vi "Controle_Manip_Main_GUI_WorkingBackup_211222.vi"() -> ()   [LabVIEW 2019] (continued)
                            n865 = control-ref of="N Step Power  Diode Current (A)"() -> (w1168:refnum<vi>)
                            n866 = control-ref of="End Power  Diod Current (A)"() -> (w1169:refnum<vi>)
                            n867 = control-ref of="Start Power Diod Current (A)"() -> (w1170:refnum<vi>)
                            n868 = property class="Bool (strict)"(reference=w1167, "Value"=FALSE) -> ()  [unwired: 1 in, 2 out]
                            n869 = control-ref of="Acquire fPow"() -> (w1174:refnum<vi>)
                            n870 = control-ref of="Save fPow"() -> (w1172:refnum<vi>)
                            n871 = Build Array(w1174, w1172, w1170, w1169, w1168) -> (w1173:refnum<vi>[])
                            n872 = call "Enable&Disable_Controls.vi"("Enum"=enum16{"Enabled", "Disabled", "Disabled&Grayed"}."Enabled", "References"=w1173) -> ()  [unwired: 1 in]
                            n873 = property on="Elapsed (s)" class="DigNum (strict)"("Visible"=FALSE) -> ()  [unwired: 2 in, 2 out]
                            n874 = local read "Auto< ?"() -> (w1162:bool)
                            n875 = control-ref of="Save fPow"() -> (w1164:refnum<vi>)
                            n876 = case shown="True" w1162 {
                              tunnel: [TRUE FALSE] -> w1161
                              frame False {
                              }
                              frame True {
                              }
                            }
                            n877 = control-ref of="MasterStop"() -> (w1159:refnum<vi>)
                            n878 = control-ref of="MasterPause"() -> (w1160:refnum<vi>)
                            n879 = control-ref of="ExperimentStopped?"() -> (w1158:refnum<vi>)
                            n880 = call "CheckStopAndReset.vi"("ExperimentStopped?"=w1158, "MasterStop"=w1159, "MasterPause"=w1160) -> ()
                            n881 = control-ref of="Acquire fPow"() -> (w1165:refnum<vi>)
                            n882 = property class="Bool (strict)"(reference=w1165, "Visible"=TRUE) -> ()  [unwired: 1 in, 2 out]
                            n883 = property class="Bool (strict)"(reference=w1164, "Visible"=w1161) -> ()  [unwired: 1 in, 2 out]
                            n884 = property on="CCD 2D Image Main" class="IntGraph (strict)"("Visible"=TRUE) -> ()  [unwired: 2 in, 2 out]
                            n885 = property on="CCD 1D Spectrum Main" class="XYGraph (strict)"("Visible"=FALSE) -> ()  [unwired: 2 in, 2 out]
                          }
                        }
                      }
                      frame "Fast Acq" {
                        n886 = stacked-sequence {
                          frame #0 {
                            w1177 = AcqMode."Spectrum" ("Acq Mode")
                            # "set port to CCD if not already"
                            n887 = property on="Acq Mode" class="Enum (strict)"() -> ("Value"=w1179:T3)  [unwired: 2 in, 2 out]
                            n888 = Not Equal?(x=w1179, y=w1177) -> (x != y?=w1178:bool)
                            n889 = case shown="True" w1178 {
                              tunnel: w1177 -> [_ w1181]
                              frame False {
                              }
                              frame True {
                                w1180 = T33 4 items=["None"=1, "SideEntrance"=2, "FrontEntrance"=3, "SideExit"=5, "FrontExit"=4] ("Exit Port Location")
                                n890 = local read "LightField Automation error out"() -> (w1191:errorcluster)
                                n891 = local read "LightField Automation out"() -> (w1190:refnum<class "LightField Automation.lvclass">)
                                n892 = property on="Acq Mode" class="Enum (strict)"("Value"=w1181) -> ()  [unwired: 2 in, 2 out]
                                n893 = call "spec_SetOpticalExitPort.vi"("error in (no error)"=w1191, "Exit Port Location"=w1180, "LightField Automation in"=w1190) -> ("error out"=w1183:errorcluster, "LightField Automation out"=w1182:refnum<class "LightField Automation.lvclass">)  [unwired: 7 in]
                                n894 = call "spec_GetCenterWavelength.vi"("error in (no error)"=w1183, "LightField Automation in"=w1182) -> ("error out"=w1186:errorcluster, "Center Wavelength"=w1184:dbl, "LightField Automation out"=w1185:refnum<class "LightField Automation.lvclass">)  [unwired: 7 in]
                                n895 = local write "Exit mirror"(w1180) -> ()
                                n896 = local write "Center Wavelength (nm)"(w1184) -> ()
                                n897 = call "spec_getCalibration.vi"("error in (no error)"=w1186, "LightField Automation in"=w1185) -> ("error out"=w1189:errorcluster, "ColumnCalibration"=w1187:dbl[], "LightField Automation out"=w1188:refnum<class "LightField Automation.lvclass">)  [unwired: 7 in]
                                n898 = local write "Wavelength calibration"(w1187) -> ()
                                n899 = local write "LightField Automation error out"(w1189) -> ()
                                n900 = local write "LightField Automation out"(w1188) -> ()
                              }
                            }
                          }
                          frame #1 {
                            # "background if none"
                            n901 = local read "Background taken?"() -> (w1192:bool)
                            n902 = case shown="False" w1192 {
                              frame False {
                                n903 = stacked-sequence {
                                tunnel: [_ _ w1238] -> w1193
                                frame #0 {
                                n904 = property on="CCD 1D Spectrum Main" class="XYGraph (strict)"("YScale.Offset"=0.0 ("Y Scale.Offset and Multiplier:Offset")) -> ()  [unwired: 2 in, 2 out]
                                }
                                frame #1 {
                                # "make sure shutter is closed"
                                n905 = local read "KCube Shutter On?"() -> (w1224:bool)
                                n906 = control-ref of="Shutter Ctrls"() -> (w1228:refnum<vi>)
                                n907 = property class="Ring (strict)"(reference=w1228) -> ("Value"=w1227:u16)  [unwired: 1 in, 2 out]
                                n908 = control-ref of="KCube Shutter Device Reference"() -> (w1229:refnum<vi>)
                                n909 = Equal?(x=w1227, y=u16 0) -> (x = y?=w1225:bool)
                                n910 = case shown="False" w1225 {
                                tunnel: w1229 -> [w1232 _]
                                tunnel: w1228 -> [w1231 _]
                                tunnel: w1224 -> [w1230 _]
                                frame False {
                                n911 = call "Shutter.vi"("KCube Shutter Device Reference 2"=w1232, "Shutter Ctrls 2"=w1231, "Shutter on?"=w1230) -> ()
                                }
                                frame True {
                                }
                                }
                                }
                                frame #2 {
                                # "acquire"
                                n912 = local read "LightField Automation error out"() -> (w1236:errorcluster)
                                n913 = local read "LightField Automation out"() -> (w1237:refnum<class "LightField Automation.lvclass">)
                                n914 = local read "Accumulations"() -> (w1233:dbl)
                                n915 = call "LFA_Capture.vi"("error in (no error)"=w1236, "Frames"=w1233, "LightField Automation in"=w1237) -> ("error out"=w1235:errorcluster, "Data"=w1238:T26, "LightField Automation out"=w1234:refnum<class "LightField Automation.lvclass">)  [unwired: 6 in]
                                n916 = local write "LightField Automation error out"(w1235) -> ()
                                n917 = local write "LightField Automation out"(w1234) -> ()
                                }
                                }
                                n918 = local read "Acq Mode"() -> (w1194:T3)
                                n919 = case shown="\"Spectrum\", Default" w1194 {
                                selector: w1194 -> [w1195 w1213]
                                tunnel: w1193 -> [w1196 w1214]
                                frame "Spectrum", Default {
                                n920 = stacked-sequence {
                                tunnel: w1196 -> [_ w1207 _ _]
                                tunnel: w1195 -> [_ w1205 _ _]
                                frame #0 {
                                n921 = property on="CCD 2D Image Main" class="IntGraph (strict)"("Visible"=FALSE) -> ()  [unwired: 2 in, 2 out]
                                n922 = property on="CCD 1D Spectrum Main" class="XYGraph (strict)"("Visible"=TRUE) -> ()  [unwired: 2 in, 2 out]
                                }
                                frame #1 {
                                n923 = local read "Wavelength calibration"() -> (w1204:dbl[])
                                n924 = local read "CCD ROI"() -> (w1200:T20)
                                n925 = Divide(x=1239.842, y=w1204) -> (x/y=w1202:dbl[])
                                n926 = call "PrepareData4Graph.vi"("Wavelength nm"=w1202, "DataLF"=w1207, "CCD ROI"=w1200, "AcqMode"=w1205, "Data type"=T30."Spectre") -> ("Spectrum"=w1206:cluster{"Array 2":dbl[], "Array":dbl[]}, "PLInt out"=w1199:dbl[])  [unwired: 2 in, 2 out]
                                n927 = local write "CCD 1D Spectrum Main"(w1206) -> ()
                                n928 = local write "BackgroundSpec"(w1199) -> ()
                                }
                                frame #2 {
                                n929 = local read "BackgroundSpec"() -> (w1208:dbl[])
                                n930 = call-poly <vilib>:"Mean.vi"("X"=w1208) -> ("mean"=w1210:dbl)  [unwired: 1 out]
                                n931 = Negate(x=w1210) -> (-x=w1209:dbl)
                                n932 = property on="CCD 1D Spectrum Main" class="XYGraph (strict)"("YScale.Offset"=w1209) -> ()  [unwired: 2 in, 2 out]
                                }
                                frame #3 {
                                n933 = local write "Background taken?"(TRUE ("Background taken?")) -> ()
                                n934 = property on="Background substract" class="Enum (strict)"("Value"=enum16{"None", "Shutter"}."None" ("Background substract")) -> ()  [unwired: 2 in, 2 out]
                                }
                                }
                                }
                                frame "Image" {
                                n935 = stacked-sequence {
                                tunnel: w1214 -> [_ w1222]
                                tunnel: w1213 -> [_ w1220]
                                frame #0 {
                                n936 = property on="CCD 1D Spectrum Main" class="XYGraph (strict)"("Visible"=FALSE) -> ()  [unwired: 2 in, 2 out]
                                n937 = property on="CCD 2D Image Main" class="IntGraph (strict)"("Visible"=TRUE) -> ()  [unwired: 2 in, 2 out]
                                }
                                frame #1 {
                                n938 = local read "Wavelength calibration"() -> (w1221:dbl[])
                                n939 = local read "CCD ROI"() -> (w1217:T20)
                                n940 = call "PrepareData4Graph.vi"("Wavelength nm"=w1221, "DataLF"=w1222, "CCD ROI"=w1217, "AcqMode"=w1220, "Data type"=T30."Spectre") -> ("Intensity Graph"=w1219:dbl[][])  [unwired: 2 in, 3 out]
                                n941 = local write "CCD 2D Image Main"(w1219) -> ()
                                }
                                }
                                }
                                }
                              }
                              frame True {
                              }
                            }
                          }
                          frame #2 {
                            # "\"measurement\""
                            n942 = stacked-sequence {
                              frame #0 {
                                # "open shutter if closed"
                                n943 = control-ref of="Shutter Ctrls"() -> (w1240:refnum<vi>)
                                n944 = property class="Ring (strict)"(reference=w1240) -> ("Value"=w1242:u16)  [unwired: 1 in, 2 out]
                                n945 = local read "KCube Shutter On?"() -> (w1245:bool)
                                n946 = control-ref of="KCube Shutter Device Reference"() -> (w1241:refnum<vi>)
                                n947 = property on="Experiment Graph Controls" class="TabCtl (strict)"("Value"=T25."Spectrum" ("Experiment Graph Controls")) -> ()  [unwired: 2 in, 2 out]
                                n948 = Equal?(x=w1242, y=u16 0) -> (x = y?=w1244:bool)
                                n949 = case shown="True" w1244 {
                                tunnel: w1241 -> [_ w1248]
                                tunnel: w1240 -> [_ w1247]
                                tunnel: w1245 -> [_ w1246]
                                frame False {
                                }
                                frame True {
                                n950 = call "Shutter.vi"("KCube Shutter Device Reference 2"=w1248, "Shutter Ctrls 2"=w1247, "Shutter on?"=w1246) -> ()
                                }
                                }
                              }
                              frame #1 {
                                # "set CCD ROI and acquire"
                                n951 = local read "LightField Automation error out"() -> (w1256:errorcluster)
                                n952 = local read "LightField Automation out"() -> (w1257:refnum<class "LightField Automation.lvclass">)
                                n953 = local read "CCD ROI"() -> (w1255:T20)
                                n954 = local read "Accumulations"() -> (w1252:dbl)
                                n955 = call "Adv_SetROI.vi"("error in (no error)"=w1256, "ROI"=w1255, "LightField Automation in"=w1257) -> ("error out"=w1253:errorcluster, "LightField Automation out"=w1254:refnum<class "LightField Automation.lvclass">)  [unwired: 7 in]
                                n956 = call "LFA_Capture.vi"("error in (no error)"=w1253, "Frames"=w1252, "LightField Automation in"=w1254) -> ("error out"=w1250:errorcluster, "Data"=w1249:T26, "LightField Automation out"=w1251:refnum<class "LightField Automation.lvclass">)  [unwired: 6 in]
                                n957 = local write "LightField Automation out"(w1251) -> ()
                                n958 = local write "LightField Automation error out"(w1250) -> ()
                                n959 = local write "Data"(w1249) -> ()
                              }
                              frame #2 {
                                # "close shutter"
                                n960 = local read "KCube Shutter On?"() -> (w1260:bool)
                                n961 = control-ref of="KCube Shutter Device Reference"() -> (w1259:refnum<vi>)
                                n962 = control-ref of="Shutter Ctrls"() -> (w1258:refnum<vi>)
                                n963 = call "Shutter.vi"("KCube Shutter Device Reference 2"=w1259, "Shutter Ctrls 2"=w1258, "Shutter on?"=w1260) -> ()
                              }
                              frame #3 {
                                # "Show data accordingly"
                                n964 = local read "Acq Mode"() -> (w1262:T3)
                                n965 = local read "Data"() -> (w1261:T26)
                                n966 = case shown="\"Spectrum\", Default" w1262 {
                                selector: w1262 -> [w1263 w1282]
                                tunnel: w1261 -> [w1264 w1283]
                                frame "Spectrum", Default {
                                n967 = stacked-sequence {
                                tunnel: w1264 -> [_ w1280 _]
                                tunnel: w1263 -> [_ w1278 _]
                                frame #0 {
                                n968 = property on="CCD 1D Spectrum Main" class="XYGraph (strict)"("Visible"=TRUE) -> ()  [unwired: 2 in, 2 out]
                                n969 = property on="CCD 2D Image Main" class="IntGraph (strict)"("Visible"=FALSE) -> ()  [unwired: 2 in, 2 out]
                                }
                                frame #1 {
                                n970 = local read "Wavelength calibration"() -> (w1277:dbl[])
                                n971 = local read "CCD ROI"() -> (w1273:T20)
                                n972 = Divide(x=1239.842, y=w1277) -> (x/y=w1275:dbl[])
                                n973 = call "PrepareData4Graph.vi"("Wavelength nm"=w1275, "DataLF"=w1280, "CCD ROI"=w1273, "AcqMode"=w1278, "Data type"=T30."Spectre") -> ("Spectrum"=w1279:cluster{"Array 2":dbl[], "Array":dbl[]}, "PLInt out"=w1272:dbl[])  [unwired: 2 in, 2 out]
                                n974 = local read "Excitation Power (uW)"() -> (w1269:dbl)
                                n975 = local write "CCD 1D Spectrum Main"(w1279) -> ()
                                n976 = local read "Acq Time (ms)"() -> (w1270:dbl)
                                n977 = local read "BackgroundSpec"() -> (w1268:dbl[])
                                n978 = local read "Display Mode"() -> (w1267:u16)
                                n979 = control-ref of="Cnts"() -> (w1271:refnum<vi>)
                                n980 = call "2Cnts.vi"("Array Background"=w1268, "Pow W"=w1269, "AcqTime ms"=w1270, "Cnts Ref"=w1271, "Display Mode"=w1267, "Array"=w1272) -> ()  [unwired: 1 out]
                                }
                                frame #2 {
                                n981 = property on="Full scale" class="Bool (strict)"("Val(Sgnl)"=TRUE ("Value (Signaling)")) -> ()  [unwired: 2 in, 2 out]
                                }
                                }
                                }
                                frame "Image" {
                                n982 = stacked-sequence {
                                tunnel: w1283 -> [_ w1291]
                                tunnel: w1282 -> [_ w1289]
                                frame #0 {
                                n983 = property on="CCD 1D Spectrum Main" class="XYGraph (strict)"("Visible"=FALSE) -> ()  [unwired: 2 in, 2 out]
                                n984 = property on="CCD 2D Image Main" class="IntGraph (strict)"("Visible"=TRUE) -> ()  [unwired: 2 in, 2 out]
                                }
                                frame #1 {
                                n985 = local read "Wavelength calibration"() -> (w1290:dbl[])
                                n986 = local read "CCD ROI"() -> (w1286:T20)
                                n987 = call "PrepareData4Graph.vi"("Wavelength nm"=w1290, "DataLF"=w1291, "CCD ROI"=w1286, "AcqMode"=w1289, "Data type"=T30."Spectre") -> ("Intensity Graph"=w1288:dbl[][])  [unwired: 2 in, 3 out]
                                n988 = local write "CCD 2D Image Main"(w1288) -> ()
                                }
                                }
                                }
                                }
                              }
                            }
                          }
                        }
                      }
                      frame "Acquire Custom Diode Spectrum" {
                        n989 = stacked-sequence {
                          frame #0 {
                            # "change exit slit to APD if needed"
                            n990 = local read "Spectrum Custom Mode"() -> (w1293:u16)
                            n991 = case shown="3" w1293 {
                              frame 0, Default {
                                n992 = control-ref of="Accumulations"() -> (w1300:refnum<vi>)
                                n993 = control-ref of="CCD ROI"() -> (w1301:refnum<vi>)
                                n994 = control-ref of="Exposure Time (ms)"() -> (w1302:refnum<vi>)
                                n995 = stacked-sequence {
                                tunnel: u16 5 ("NewVal") -> [w1304 w1309 _]
                                tunnel: [_ w1308 _] -> w1298
                                tunnel: [_ w1307 _] -> w1297
                                frame #0 {
                                n996 = control-ref of="Exit mirror"() -> (w1303:refnum<vi>)
                                n997 = property class="Ring (strict)"(reference=w1303, "Value"=w1304) -> ()  [unwired: 1 in, 2 out]
                                n998 = Build Array(w1303) -> (w1306:refnum<vi>[])
                                n999 = call "Enable&Disable_Controls.vi"("Enum"=enum16{"Enabled", "Disabled", "Disabled&Grayed"}."Disabled&Grayed", "References"=w1306) -> ()  [unwired: 1 in]
                                }
                                frame #1 {
                                n1000 = local read "LightField Automation error out"() -> (w1317:errorcluster)
                                n1001 = case shown="4, Default" w1309 {
                                tunnel: [enum16{"Enabled", "Disabled", "Disabled&Grayed"}."Disabled&Grayed" ("Enum") enum16{"Enabled", "Disabled", "Disabled&Grayed"}."Enabled" ("Enum")] -> w1308
                                tunnel: [AcqMode."APD 1" ("Acq Mode") AcqMode."Spectrum" ("Acq Mode")] -> w1307
                                frame 5 {
                                }
                                frame 4, Default {
                                }
                                }
                                n1002 = local read "LightField Automation out"() -> (w1316:refnum<class "LightField Automation.lvclass">)
                                n1003 = call "spec_GetOpticalExitPort.vi"("error in (no error)"=w1317, "LightField Automation in"=w1316) -> ("error out"=w1314:errorcluster, "Exit Port Location"=w1313:T33, "LightField Automation out"=w1315:refnum<class "LightField Automation.lvclass">)  [unwired: 7 in]
                                n1004 = Equal?(x=w1313, y=w1309) -> (x = y?=w1312:bool)
                                n1005 = case shown="False" w1312 {
                                tunnel: w1315 -> [w1338 w1340]
                                tunnel: w1314 -> [w1337 w1339]
                                tunnel: w1309 -> [w1336 _]
                                tunnel: [w1329 w1340] -> w1311
                                tunnel: [w1328 w1339] -> w1310
                                frame False {
                                n1006 = call "spec_SetOpticalExitPort.vi"("error in (no error)"=w1337, "Exit Port Location"=w1336, "LightField Automation in"=w1338) -> ("error out"=w1331:errorcluster, "LightField Automation out"=w1330:refnum<class "LightField Automation.lvclass">)  [unwired: 7 in]
                                n1007 = call "spec_GetCenterWavelength.vi"("error in (no error)"=w1331, "LightField Automation in"=w1330) -> ("error out"=w1334:errorcluster, "Center Wavelength"=w1332:dbl, "LightField Automation out"=w1333:refnum<class "LightField Automation.lvclass">)  [unwired: 7 in]
                                n1008 = local write "Center Wavelength (nm)"(w1332) -> ()
                                n1009 = call "spec_getCalibration.vi"("error in (no error)"=w1334, "LightField Automation in"=w1333) -> ("error out"=w1328:errorcluster, "ColumnCalibration"=w1335:dbl[], "LightField Automation out"=w1329:refnum<class "LightField Automation.lvclass">)  [unwired: 7 in]
                                n1010 = local write "Wavelength calibration"(w1335) -> ()
                                n1011 = property on="Exit mirror" class="Ring (strict)"() -> ("RingText.Text"=w1324:string)  [unwired: 2 in, 2 out]
                                n1012 = local read "Log file"() -> (w1327:string)
                                n1013 = Concatenate Strings("Exit mirror set to " ("Add to log file"), w1324) -> (w1325:string)
                                n1014 = call "Write2LogFile.vi"("Add to log file"=w1325, "Log file before"=w1327, "Checkbox"=FALSE) -> ("Log file after"=w1326:string)
                                n1015 = local write "Log file"(w1326) -> ()
                                }
                                frame True {
                                }
                                }
                                n1016 = local write "LightField Automation error out"(w1310) -> ()
                                n1017 = local write "LightField Automation out"(w1311) -> ()
                                }
                                frame #2 {
                                n1018 = control-ref of="Exit mirror"() -> (w1343:refnum<vi>)
                                n1019 = Build Array(w1343) -> (w1342:refnum<vi>[])
                                n1020 = call "Enable&Disable_Controls.vi"("Enum"=enum16{"Enabled", "Disabled", "Disabled&Grayed"}."Enabled", "References"=w1342) -> ()  [unwired: 1 in]
                                }
                                }
                                n1021 = Build Array(w1300, w1301, w1302) -> (w1299:refnum<vi>[])
                                n1022 = call "Enable&Disable_Controls.vi"("Enum"=w1298, "References"=w1299) -> ()  [unwired: 1 in]
                                n1023 = property on="Acq Mode" class="Enum (strict)"("Value"=w1297) -> ()  [unwired: 2 in, 2 out]
                              }
                              frame 1 {
                                n1024 = control-ref of="Accumulations"() -> (w1348:refnum<vi>)
                                n1025 = control-ref of="CCD ROI"() -> (w1349:refnum<vi>)
                                n1026 = control-ref of="Exposure Time (ms)"() -> (w1350:refnum<vi>)
                                n1027 = stacked-sequence {
                                tunnel: u16 5 ("NewVal") -> [w1352 w1357 _]
                                tunnel: [_ w1356 _] -> w1346
                                tunnel: [_ w1355 _] -> w1345
                                frame #0 {
                                n1028 = control-ref of="Exit mirror"() -> (w1351:refnum<vi>)
                                n1029 = property class="Ring (strict)"(reference=w1351, "Value"=w1352) -> ()  [unwired: 1 in, 2 out]
                                n1030 = Build Array(w1351) -> (w1354:refnum<vi>[])
                                n1031 = call "Enable&Disable_Controls.vi"("Enum"=enum16{"Enabled", "Disabled", "Disabled&Grayed"}."Disabled&Grayed", "References"=w1354) -> ()  [unwired: 1 in]
                                }
                                frame #1 {
                                n1032 = local read "LightField Automation error out"() -> (w1365:errorcluster)
                                n1033 = case shown="5" w1357 {
                                tunnel: [enum16{"Enabled", "Disabled", "Disabled&Grayed"}."Disabled&Grayed" ("Enum") enum16{"Enabled", "Disabled", "Disabled&Grayed"}."Enabled" ("Enum")] -> w1356
                                tunnel: [AcqMode."APD 1" ("Acq Mode") AcqMode."Spectrum" ("Acq Mode")] -> w1355
                                frame 5 {
                                }
                                frame 4, Default {
                                }
                                }
                                n1034 = local read "LightField Automation out"() -> (w1364:refnum<class "LightField Automation.lvclass">)
                                n1035 = call "spec_GetOpticalExitPort.vi"("error in (no error)"=w1365, "LightField Automation in"=w1364) -> ("error out"=w1362:errorcluster, "Exit Port Location"=w1361:T33, "LightField Automation out"=w1363:refnum<class "LightField Automation.lvclass">)  [unwired: 7 in]
                                n1036 = Equal?(x=w1361, y=w1357) -> (x = y?=w1360:bool)
                                n1037 = case shown="False" w1360 {
                                tunnel: w1363 -> [w1386 w1388]
                                tunnel: w1362 -> [w1385 w1387]
                                tunnel: w1357 -> [w1384 _]
                                tunnel: [w1377 w1388] -> w1359
                                tunnel: [w1376 w1387] -> w1358
                                frame False {
                                n1038 = call "spec_SetOpticalExitPort.vi"("error in (no error)"=w1385, "Exit Port Location"=w1384, "LightField Automation in"=w1386) -> ("error out"=w1379:errorcluster, "LightField Automation out"=w1378:refnum<class "LightField Automation.lvclass">)  [unwired: 7 in]
                                n1039 = call "spec_GetCenterWavelength.vi"("error in (no error)"=w1379, "LightField Automation in"=w1378) -> ("error out"=w1382:errorcluster, "Center Wavelength"=w1380:dbl, "LightField Automation out"=w1381:refnum<class "LightField Automation.lvclass">)  [unwired: 7 in]
                                n1040 = local write "Center Wavelength (nm)"(w1380) -> ()
                                n1041 = call "spec_getCalibration.vi"("error in (no error)"=w1382, "LightField Automation in"=w1381) -> ("error out"=w1376:errorcluster, "ColumnCalibration"=w1383:dbl[], "LightField Automation out"=w1377:refnum<class "LightField Automation.lvclass">)  [unwired: 7 in]
                                n1042 = local write "Wavelength calibration"(w1383) -> ()
                                n1043 = property on="Exit mirror" class="Ring (strict)"() -> ("RingText.Text"=w1372:string)  [unwired: 2 in, 2 out]
                                n1044 = local read "Log file"() -> (w1375:string)
                                n1045 = Concatenate Strings("Exit mirror set to " ("Add to log file"), w1372) -> (w1373:string)
                                n1046 = call "Write2LogFile.vi"("Add to log file"=w1373, "Log file before"=w1375, "Checkbox"=FALSE) -> ("Log file after"=w1374:string)
                                n1047 = local write "Log file"(w1374) -> ()
                                }
                                frame True {
                                }
                                }
                                n1048 = local write "LightField Automation error out"(w1358) -> ()
                                n1049 = local write "LightField Automation out"(w1359) -> ()
                                }
                                frame #2 {
                                n1050 = control-ref of="Exit mirror"() -> (w1391:refnum<vi>)
                                n1051 = Build Array(w1391) -> (w1390:refnum<vi>[])
                                n1052 = call "Enable&Disable_Controls.vi"("Enum"=enum16{"Enabled", "Disabled", "Disabled&Grayed"}."Enabled", "References"=w1390) -> ()  [unwired: 1 in]
                                }
                                }
                                n1053 = Build Array(w1348, w1349, w1350) -> (w1347:refnum<vi>[])
                                n1054 = call "Enable&Disable_Controls.vi"("Enum"=w1346, "References"=w1347) -> ()  [unwired: 1 in]
                                n1055 = property on="Acq Mode" class="Enum (strict)"("Value"=w1345) -> ()  [unwired: 2 in, 2 out]
                              }
                              frame 3 {
                                n1056 = control-ref of="Accumulations"() -> (w1396:refnum<vi>)
                                n1057 = control-ref of="CCD ROI"() -> (w1397:refnum<vi>)
                                n1058 = control-ref of="Exposure Time (ms)"() -> (w1398:refnum<vi>)
                                n1059 = stacked-sequence {
                                tunnel: u16 5 ("NewVal") -> [w1400 w1405 _]
                                tunnel: [_ w1404 _] -> w1394
                                tunnel: [_ w1403 _] -> w1393
                                frame #0 {
                                n1060 = control-ref of="Exit mirror"() -> (w1399:refnum<vi>)
                                n1061 = property class="Ring (strict)"(reference=w1399, "Value"=w1400) -> ()  [unwired: 1 in, 2 out]
                                n1062 = Build Array(w1399) -> (w1402:refnum<vi>[])
                                n1063 = call "Enable&Disable_Controls.vi"("Enum"=enum16{"Enabled", "Disabled", "Disabled&Grayed"}."Disabled&Grayed", "References"=w1402) -> ()  [unwired: 1 in]
                                }
                                frame #1 {
                                n1064 = local read "LightField Automation error out"() -> (w1413:errorcluster)
                                n1065 = case shown="4, Default" w1405 {
                                tunnel: [enum16{"Enabled", "Disabled", "Disabled&Grayed"}."Disabled&Grayed" ("Enum") enum16{"Enabled", "Disabled", "Disabled&Grayed"}."Enabled" ("Enum")] -> w1404
                                tunnel: [AcqMode."APD 1+2" ("Acq Mode") AcqMode."Spectrum" ("Acq Mode")] -> w1403
                                frame 5 {
                                }
                                frame 4, Default {
                                }
                                }
                                n1066 = local read "LightField Automation out"() -> (w1412:refnum<class "LightField Automation.lvclass">)
                                n1067 = call "spec_GetOpticalExitPort.vi"("error in (no error)"=w1413, "LightField Automation in"=w1412) -> ("error out"=w1410:errorcluster, "Exit Port Location"=w1409:T33, "LightField Automation out"=w1411:refnum<class "LightField Automation.lvclass">)  [unwired: 7 in]
                                n1068 = Equal?(x=w1409, y=w1405) -> (x = y?=w1408:bool)
                                n1069 = case shown="False" w1408 {
                                tunnel: w1411 -> [w1434 w1436]
                                tunnel: w1410 -> [w1433 w1435]
                                tunnel: w1405 -> [w1432 _]
                                tunnel: [w1425 w1436] -> w1407
                                tunnel: [w1424 w1435] -> w1406
                                frame False {
                                n1070 = call "spec_SetOpticalExitPort.vi"("error in (no error)"=w1433, "Exit Port Location"=w1432, "LightField Automation in"=w1434) -> ("error out"=w1427:errorcluster, "LightField Automation out"=w1426:refnum<class "LightField Automation.lvclass">)  [unwired: 7 in]
                                n1071 = call "spec_GetCenterWavelength.vi"("error in (no error)"=w1427, "LightField Automation in"=w1426) -> ("error out"=w1430:errorcluster, "Center Wavelength"=w1428:dbl, "LightField Automation out"=w1429:refnum<class "LightField Automation.lvclass">)  [unwired: 7 in]
                                n1072 = local write "Center Wavelength (nm)"(w1428) -> ()
                                n1073 = call "spec_getCalibration.vi"("error in (no error)"=w1430, "LightField Automation in"=w1429) -> ("error out"=w1424:errorcluster, "ColumnCalibration"=w1431:dbl[], "LightField Automation out"=w1425:refnum<class "LightField Automation.lvclass">)  [unwired: 7 in]
                                n1074 = local write "Wavelength calibration"(w1431) -> ()
                                n1075 = property on="Exit mirror" class="Ring (strict)"() -> ("RingText.Text"=w1420:string)  [unwired: 2 in, 2 out]
                                n1076 = local read "Log file"() -> (w1423:string)
                                n1077 = Concatenate Strings("Exit mirror set to " ("Add to log file"), w1420) -> (w1421:string)
                                n1078 = call "Write2LogFile.vi"("Add to log file"=w1421, "Log file before"=w1423, "Checkbox"=FALSE) -> ("Log file after"=w1422:string)
                                n1079 = local write "Log file"(w1422) -> ()
                                }
                                frame True {
                                }
                                }
                                n1080 = local write "LightField Automation error out"(w1406) -> ()
                                n1081 = local write "LightField Automation out"(w1407) -> ()
                                }
                                frame #2 {
                                n1082 = control-ref of="Exit mirror"() -> (w1439:refnum<vi>)
                                n1083 = Build Array(w1439) -> (w1438:refnum<vi>[])
                                n1084 = call "Enable&Disable_Controls.vi"("Enum"=enum16{"Enabled", "Disabled", "Disabled&Grayed"}."Enabled", "References"=w1438) -> ()  [unwired: 1 in]
                                }
                                }
                                n1085 = Build Array(w1396, w1397, w1398) -> (w1395:refnum<vi>[])
                                n1086 = call "Enable&Disable_Controls.vi"("Enum"=w1394, "References"=w1395) -> ()  [unwired: 1 in]
                                n1087 = property on="Acq Mode" class="Enum (strict)"("Value"=w1393) -> ()  [unwired: 2 in, 2 out]
                              }
                              frame 2 {
                                n1088 = property on="Acq Mode" class="Enum (strict)"("Value"=AcqMode."APD 2" ("Acq Mode")) -> ()  [unwired: 2 in, 2 out]
                              }
                              frame 4 {
                                n1089 = property on="Acq Mode" class="Enum (strict)"("Value"=AcqMode."APD 2" ("Acq Mode")) -> ()  [unwired: 2 in, 2 out]
                              }
                            }
                            n1090 = local read "Scan Spectrum Cust Params"() -> (w1295:refnum<vi>[])
                            n1091 = call "Enable&Disable_Controls.vi"("Enum"=enum16{"Enabled", "Disabled", "Disabled&Grayed"}."Disabled&Grayed", "References"=w1295) -> ()  [unwired: 1 in]
                            n1092 = property on="Experiment Graph Controls" class="TabCtl (strict)"("Value"=T25."Spectrum" ("Experiment Graph Controls")) -> ()  [unwired: 2 in, 2 out]
                          }
                          frame #1 {
                            n1093 = local read "Spectrum Step Wavelength (nm)"() -> (w1449:dbl)
                            n1094 = local read "Spectrum End Wavelength (nm)"() -> (w1448:dbl)
                            n1095 = local read "Spectrum Start Wavelength (nm)"() -> (w1450:dbl)
                            n1096 = local read "Spectrum Custom Mode"() -> (w1447:u16)
                            n1097 = local read "KCube Shutter On?"() -> (w1446:bool)
                            n1098 = local read "Acq Time (ms)"() -> (w1445:dbl)
                            n1099 = Bundle("Acq Time (ms)"=w1445, "Spectrum Start Wavelength (nm)"=w1450, "Spectrum Step Wavelength (nm)"=w1449, "Spectrum End Wavelength (nm)"=w1448, "Spectrum Custom Mode"=w1447, "KCube Shutter On?"=w1446) -> (→"Scan Spectrum Cust Exp Params":T18)  [unwired: 1 in]
                            n1100 = control-ref of="MasterStop"() -> (w1443:refnum<vi>)
                            n1101 = property class="Bool (strict)"(reference=w1443, "Visible"=TRUE) -> ()  [unwired: 1 in, 2 out]
                          }
                          frame #2 {
                            n1102 = local read "Spectrum Custom Mode"() -> (w1451:u16)
                            n1103 = case shown="1" w1451 {
                              frame 0, Default {
                                # "PD1 \nScan monochromator SpectraPro HRS with photodiode at APD exit slit"
                                n1104 = control-ref of="Scan Main Progess Bar"() -> (w1455:refnum<vi>)
                                n1105 = local read "LightField Automation out"() -> (w1467:refnum<class "LightField Automation.lvclass">)
                                n1106 = local read "Photodiode handle out"() -> (w1466:refnum<visa-resource-name>)
                                n1107 = local read "LightField Automation error out"() -> (w1464:errorcluster)
                                n1108 = local read "Photodiode error out"() -> (w1465:errorcluster)
                                n1109 = control-ref of="CCD 1D Spectrum Main"() -> (w1463:refnum<vi>)
                                n1110 = control-ref of="Center Wavelength (nm)"() -> (w1461:refnum<vi>)
                                n1111 = control-ref of="Stop Spectrum Custom"() -> ()  [unwired: 1 out]
                                n1112 = control-ref of="Excitation Power (uW)"() -> (w1456:refnum<vi>)
                                n1113 = local read "Scan Spectrum Cust Exp Params"() -> (w1462:T18)
                                n1114 = control-ref of="MasterStop"() -> (w1452:refnum<vi>)
                                n1115 = call "CustomSpectrum.vi"("LightField Automation"=w1467, "Photodiode handle out"=w1466, "Stop Spectrum Custom"=w1452, "Photodiode error out"=w1465, "LightField Automation error"=w1464, "CCD 1D Spectrum Main"=w1463, "Center Wavelength (nm)"=w1461, "Scan Spectrum Progess Bar"=w1455, "Excitation Power (uW)"=w1456, "Scan Spectrum Cust Exp Params 2"=w1462) -> ("WLs"=w1454:dbl[], "PL"=w1453:dbl[], "LFA Out"=w1460:refnum<class "LightField Automation.lvclass">, "PD Out"=w1459:refnum<visa-resource-name>, "PD Error Our"=w1458:errorcluster, "LFA Error Out"=w1457:errorcluster)  [unwired: 3 in, 1 out]
                                n1116 = local write "Data PL Custom Diode Spectrum"(w1453) -> ()
                                n1117 = local write "Wavelength calibration"(w1454) -> ()
                                n1118 = local write "LightField Automation out"(w1460) -> ()
                                n1119 = local write "Photodiode handle out"(w1459) -> ()
                                n1120 = local write "LightField Automation error out"(w1457) -> ()
                                n1121 = local write "Photodiode error out"(w1458) -> ()
                              }
                              frame 1 {
                                # "APD1 Scan monochromator SpectraPro HRS and acquire APD 1"
                                n1122 = stacked-sequence {
                                frame #0 {
                                n1123 = property on="Save Custom Diode Spectrum" class="Bool (strict)"("Visible"=FALSE) -> ()  [unwired: 2 in, 2 out]
                                n1124 = local read "KCube Shutter On?"() -> (w1472:bool)
                                n1125 = control-ref of="Shutter Ctrls"() -> (w1473:refnum<vi>)
                                n1126 = control-ref of="KCube Shutter Device Reference"() -> (w1474:refnum<vi>)
                                n1127 = call "Shutter.vi"("KCube Shutter Device Reference 2"=w1474, "Shutter Ctrls 2"=w1473, "Shutter on?"=w1472) -> ()
                                n1128 = property on="CCD 1D Spectrum Main" class="XYGraph (strict)"("YScale.Offset"=0.0 ("Y Scale.Offset and Multiplier:Offset"), "YScale.Minimum"=0.0 ("Y Scale.Range:Minimum")) -> ()  [unwired: 2 in, 2 out]
                                n1129 = property on="Elapsed (s)" class="DigNum (strict)"("Visible"=TRUE) -> ()  [unwired: 2 in, 2 out]
                                }
                                frame #1 {
                                n1130 = local read "PH_Init_Data"() -> (w1486:T11)
                                n1131 = local read "PH_Settings_Params"() -> (w1485:T10)
                                n1132 = Unbundle By Name(w1486) -> ("Deviceindex"=w1483:i32)
                                n1133 = local read "PH_CFD1 level"() -> (w1480:i32)
                                n1134 = local read "PH_CFD1 zero X"() -> (w1479:i32)
                                n1135 = local read "Acq Time (ms)"() -> (w1476:dbl)
                                n1136 = local read "PH_Range No."() -> (w1478:i32)
                                n1137 = local read "PH_CFD0 level"() -> (w1482:i32)
                                n1138 = local read "PH_CFD0 zero X"() -> (w1481:i32)
                                n1139 = local read "PH_SyncDiv"() -> (w1484:enum16{"1", "2", "4", "8"})
                                n1140 = Bundle By Name(cluster=w1485, "SyncDiv"=w1484, "DeviceIndex"=w1483, "CFD0 level"=w1482, "CFD0 zero X"=w1481, "CFD1 level"=w1480, "CFD1 zero X"=w1479, "Range No."=w1478, "StopOnOverflow"=TRUE, "AcqTime (ms)"=w1476) -> (w1475:T10)
                                n1141 = local write "PH_Settings_Params"(w1475) -> ()
                                }
                                frame #2 {
                                n1142 = local read "LightField Automation error out"() -> (w1495:errorcluster)
                                n1143 = local read "Scan Spectrum Cust Exp Params"() -> (w1494:T18)
                                n1144 = control-ref of="Center Wavelength (nm)"() -> (w1497:refnum<vi>)
                                n1145 = control-ref of="CCD 1D Spectrum Main"() -> (w1498:refnum<vi>)
                                n1146 = local read "LightField Automation out"() -> (w1496:refnum<class "LightField Automation.lvclass">)
                                n1147 = local read "PH_Settings_Params"() -> (w1492:T10)
                                n1148 = local read "PH_Init_Data"() -> (w1493:T11)
                                n1149 = control-ref of="Stop Spectrum Custom"() -> ()  [unwired: 1 out]
                                n1150 = control-ref of="Scan Main Progess Bar"() -> (w1499:refnum<vi>)
                                n1151 = control-ref of="MasterStop"() -> (w1487:refnum<vi>)
                                n1152 = call "CustomAPDSpectrum.vi"("LightField Automation"=w1496, "PH_Init_Data"=w1493, "PH_Settings_Params"=w1492, "Stop Spectrum Custom"=w1487, "LightField Automation error"=w1495, "CCD 1D Spectrum Main"=w1498, "Center Wavelength (nm)"=w1497, "Scan Spectrum Progess Bar"=w1499, "Scan Spectrum Cust Exp Params 2"=w1494) -> ("WLs"=w1489:dbl[], "LFA Out"=w1491:refnum<class "LightField Automation.lvclass">, "PL"=→"Data PL Custom Diode Spectrum":dbl[], "LFA Error Out"=w1490:errorcluster)  [unwired: 6 in, 1 out]
                                n1153 = local write "Wavelength calibration"(w1489) -> ()
                                n1154 = local write "LightField Automation error out"(w1490) -> ()
                                n1155 = local write "LightField Automation out"(w1491) -> ()
                                }
                                frame #3 {
                                n1156 = local read "KCube Shutter On?"() -> (w1505:bool)
                                n1157 = control-ref of="Shutter Ctrls"() -> (w1506:refnum<vi>)
                                n1158 = control-ref of="KCube Shutter Device Reference"() -> (w1507:refnum<vi>)
                                n1159 = call "Shutter.vi"("KCube Shutter Device Reference 2"=w1507, "Shutter Ctrls 2"=w1506, "Shutter on?"=w1505) -> ()
                                n1160 = property on="Full scale" class="Bool (strict)"("Val(Sgnl)"=TRUE ("Value (Signaling)")) -> ()  [unwired: 2 in, 2 out]
                                n1161 = property on="Elapsed (s)" class="DigNum (strict)"("Visible"=FALSE) -> ()  [unwired: 2 in, 2 out]
                                n1162 = local write "Background taken?"(FALSE ("Background taken?")) -> ()
                                n1163 = property on="CCD 1D Spectrum Main" class="XYGraph (strict)"("YScale.Offset"=0.0 ("Y Scale.Offset and Multiplier:Offset"), "YScale.Minimum"=0.0 ("Y Scale.Range:Minimum")) -> ()  [unwired: 2 in, 2 out]
                                }
                                }
                              }
                              frame 2 {
                                # "APD2 Scan monochromator iHR320 and acquire APD 2 // quick&dirty avant calib"
                                n1164 = stacked-sequence {
                                frame #0 {
                                w1508 = 0.0 ("Y Scale.Offset and Multiplier:Offset")
                                n1165 = property on="Elapsed (s)" class="DigNum (strict)"("Visible"=TRUE) -> ()  [unwired: 2 in, 2 out]
                                n1166 = property on="Save Custom Diode Spectrum" class="Bool (strict)"("Visible"=FALSE) -> ()  [unwired: 2 in, 2 out]
                                n1167 = local read "KCube Shutter On?"() -> (w1511:bool)
                                n1168 = control-ref of="Shutter Ctrls"() -> (w1512:refnum<vi>)
                                n1169 = control-ref of="KCube Shutter Device Reference"() -> (w1513:refnum<vi>)
                                n1170 = call "Shutter.vi"("KCube Shutter Device Reference 2"=w1513, "Shutter Ctrls 2"=w1512, "Shutter on?"=w1511) -> ()
                                n1171 = property on="CCD 1D Spectrum Main" class="XYGraph (strict)"("YScale.Offset"=w1508, "YScale.Minimum"=w1508) -> ()  [unwired: 2 in, 2 out]
                                }
                                frame #1 {
                                n1172 = local read "PH_Init_Data"() -> (w1524:T11)
                                n1173 = local read "PH_Settings_Params"() -> (w1525:T10)
                                n1174 = Unbundle By Name(w1524) -> ("Deviceindex"=w1522:i32)
                                n1175 = local read "PH_CFD1 level"() -> (w1519:i32)
                                n1176 = local read "PH_CFD1 zero X"() -> (w1518:i32)
                                n1177 = local read "Acq Time (ms)"() -> (w1516:dbl)
                                n1178 = local read "PH_Range No."() -> (w1517:i32)
                                n1179 = local read "PH_CFD0 level"() -> (w1521:i32)
                                n1180 = local read "PH_CFD0 zero X"() -> (w1520:i32)
                                n1181 = local read "PH_SyncDiv"() -> (w1523:enum16{"1", "2", "4", "8"})
                                n1182 = Bundle By Name(cluster=w1525, "SyncDiv"=w1523, "DeviceIndex"=w1522, "CFD0 level"=w1521, "CFD0 zero X"=w1520, "CFD1 level"=w1519, "CFD1 zero X"=w1518, "Range No."=w1517, "StopOnOverflow"=TRUE, "AcqTime (ms)"=w1516) -> (w1515:T10)
                                n1183 = local write "PH_Settings_Params"(w1515) -> ()
                                }
                                frame #2 {
                                n1184 = local read "Spectrum End Wavelength (nm)"() -> (w1533:dbl)
                                n1185 = local read "Spectrum Step Wavelength (nm)"() -> (w1527:dbl)
                                n1186 = local read "Spectrum Start Wavelength (nm)"() -> (w1531:dbl)
                                n1187 = Subtract(x=w1533, y=w1531) -> (x-y=w1535:dbl)
                                n1188 = Divide(x=w1535, y=w1527) -> (x/y=w1534:dbl)
                                n1189 = Increment(x=w1534) -> (x+1=w1532:dbl)
                                n1190 = for {
                                N: w1532 -> [_]
                                tunnel: w1527 -> [w1550]
                                tunnel: w1531 -> [w1549]
                                shift-right: [w1536] -> w1528
                                shift-left: dbl[] [] -> [w1544]
                                shift-right: [w1541] -> w1526
                                shift-left: dbl[] [] -> [w1545]
                                i -> [w1551]
                                stop <- w1539 stop-if-true
                                n1191 = control-ref of="MasterStop"() -> (w1538:refnum<vi>)
                                n1192 = control-ref of="Stop Spectrum Custom"() -> ()  [unwired: 1 out]
                                n1193 = Multiply(x=w1551, y=w1550) -> (x*y=w1548:dbl)
                                n1194 = Add(x=w1549, y=w1548) -> (x+y=w1540:dbl)
                                n1195 = local read "ESP300 COM Port"() -> (w1547:refnum<visa-resource-name>)
                                n1196 = stacked-sequence {
                                tunnel: w1540 -> [w1553 _ _]
                                tunnel: w1547 -> [w1561 _ _]
                                tunnel: [_ _ w1563] -> w1546
                                tunnel: w1545 -> [w1559 _ _]
                                tunnel: [w1558 _ _] -> w1541
                                frame #0 {
                                w1555 = u16 1 items=["Detection"=1, "Excitation"=2] ("HR mode")
                                n1197 = call "MotorWL2Pos.vi"("Mono2 Center WL"=w1553, "HR mode"=w1555) -> ("Mono2 Position"=w1557:dbl)
                                n1198 = control-ref of="Mono2 Motor Pos"() -> (w1560:refnum<vi>)
                                n1199 = control-ref of="Mono2 Wavelength (nm)"() -> (w1556:refnum<vi>)
                                n1200 = call "subVI_Mono2Go2Posv2.vi"("Mono2 Motor Pos"=w1560, "Mono2 Wavelength (nm)"=w1556, "HR mode"=w1555, "Postion (Unit)"=w1557, "ESP300 COM Port"=w1561) -> ()  [unwired: 2 out]
                                n1201 = Divide(x=1239.842, y=w1553) -> (x/y=w1552:dbl)
                                n1202 = Insert Into Array(array=w1559, new element=w1552) -> (w1558:dbl[])  [unwired: 1 in]
                                }
                                frame #1 {
                                n1203 = Wait (ms)(milliseconds to wait=u32 20) -> ()  [unwired: 1 out]
                                }
                                frame #2 {
                                n1204 = local read "PH_Settings_Params"() -> (w1564:T10)
                                n1205 = local read "PH_Init_Data"() -> (w1565:T11)
                                n1206 = Unbundle By Name(w1565) -> ("Initialization Error"=w1569:bool, "Calib Error"=w1568:bool, "Deviceindex"=w1567:i32)
                                n1207 = call "PH_Acq_ms.vi"("PH_Settings_Params"=w1564, "Deviceindex"=w1567, "Calib Error"=w1568, "Initialization Error"=w1569) -> ("CH1MeanRate"=w1563:dbl, "SyncMeanRate"=w1566:dbl)  [unwired: 1 out]
                                n1208 = Build Array(w1566, w1563) -> ()  [unwired: 1 out]
                                }
                                }
                                n1209 = property class="Bool (strict)"(reference=w1538) -> ("Value"=w1539:bool)  [unwired: 1 in, 2 out]
                                n1210 = control-ref of="CCD 1D Spectrum Main"() -> (w1543:refnum<vi>)
                                n1211 = Insert Into Array(array=w1544, new element=w1546) -> (w1536:dbl[])  [unwired: 1 in]
                                n1212 = call "myMaxAPDs.vi"("Array"=w1536) -> ("myMax"=w1537:dbl)
                                n1213 = Bundle(w1541, w1536) -> (w1542:cluster{dbl[], dbl[]})  [unwired: 1 in]
                                n1214 = property class="XYGraph (strict)"(reference=w1543, "Value"=w1542, "YScale.Maximum"=w1537) -> ()  [unwired: 1 in, 2 out]
                                }
                                n1215 = local write "Wavelength calibration"(w1526) -> ()
                                n1216 = local write "Data PL Custom Diode Spectrum"(w1528) -> ()
                                }
                                frame #3 {
                                n1217 = property on="Elapsed (s)" class="DigNum (strict)"("Visible"=FALSE) -> ()  [unwired: 2 in, 2 out]
                                n1218 = local read "KCube Shutter On?"() -> (w1575:bool)
                                n1219 = control-ref of="Shutter Ctrls"() -> (w1576:refnum<vi>)
                                n1220 = property on="CCD 1D Spectrum Main" class="XYGraph (strict)"("YScale.Offset"=0.0 ("Y Scale.Offset and Multiplier:Offset"), "YScale.Minimum"=0.0 ("Y Scale.Range:Minimum")) -> ()  [unwired: 2 in, 2 out]
                                n1221 = control-ref of="KCube Shutter Device Reference"() -> (w1577:refnum<vi>)
                                n1222 = call "Shutter.vi"("KCube Shutter Device Reference 2"=w1577, "Shutter Ctrls 2"=w1576, "Shutter on?"=w1575) -> ()
                                n1223 = local write "Background taken?"(FALSE ("Background taken?")) -> ()
                                n1224 = property on="Full scale" class="Bool (strict)"("Val(Sgnl)"=TRUE ("Value (Signaling)")) -> ()  [unwired: 2 in, 2 out]
                                }
                                }
                              }
                              frame 3 {
                                # "ADP1&2 Scan both monochromators synchronously and both APD outputs"
                              }
                              frame 4 {
                                # "PD2 Scan monochromator iHR320 with photodiode at APD exit slit"
                                n1225 = stacked-sequence {
                                frame #0 {
                                n1226 = property on="Elapsed (s)" class="DigNum (strict)"("Visible"=TRUE) -> ()  [unwired: 2 in, 2 out]
                                n1227 = property on="Save Custom Diode Spectrum" class="Bool (strict)"("Visible"=FALSE) -> ()  [unwired: 2 in, 2 out]
                                n1228 = local read "KCube Shutter On?"() -> (w1580:bool)
                                n1229 = control-ref of="Shutter Ctrls"() -> (w1581:refnum<vi>)
                                n1230 = control-ref of="KCube Shutter Device Reference"() -> (w1582:refnum<vi>)
                                n1231 = call "Shutter.vi"("KCube Shutter Device Reference 2"=w1582, "Shutter Ctrls 2"=w1581, "Shutter on?"=w1580) -> ()
                                }
                                frame #1 {
                                n1232 = local read "PH_Init_Data"() -> (w1593:T11)
                                n1233 = local read "PH_Settings_Params"() -> (w1594:T10)
                                n1234 = local read "PH_CFD1 level"() -> (w1588:i32)
                                n1235 = local read "PH_CFD1 zero X"() -> (w1587:i32)
                                n1236 = local read "Acq Time (ms)"() -> (w1585:dbl)
                                n1237 = local read "PH_Range No."() -> (w1586:i32)
                                n1238 = Unbundle By Name(w1593) -> ("Deviceindex"=w1591:i32)
                                n1239 = local read "PH_CFD0 level"() -> (w1590:i32)
                                n1240 = local read "PH_CFD0 zero X"() -> (w1589:i32)
                                n1241 = local read "PH_SyncDiv"() -> (w1592:enum16{"1", "2", "4", "8"})
                                n1242 = Bundle By Name(cluster=w1594, "SyncDiv"=w1592, "DeviceIndex"=w1591, "CFD0 level"=w1590, "CFD0 zero X"=w1589, "CFD1 level"=w1588, "CFD1 zero X"=w1587, "Range No."=w1586, "StopOnOverflow"=TRUE, "AcqTime (ms)"=w1585) -> (w1584:T10)
                                n1243 = local write "PH_Settings_Params"(w1584) -> ()